vi "FlexMag - 23-03-2023.vi"() -> ()   [LabVIEW 2018] (continued)
                                }
                                frame #1 {
                                n20432 = local read "abort ch2"() -> (w24637:bool)
                                n20433 = case shown="False" w24637 {
                                frame False {
                                n20434 = local read "coating start"() -> (w24638:bool)
                                n20435 = case shown="True" w24638 {
                                frame False {
                                }
                                frame True {
                                n20436 = while {
                                i -> [w24644]
                                stop <- w24646 stop-if-true
                                n20437 = Greater Or Equal?(x=w24644, y=50) -> (x >= y?=w24645:bool)
                                n20438 = case shown="True" w24645 {
                                frame False {
                                }
                                frame True {
                                n20439 = local write "Warning Message"("Automatic Coating Process is canceled !\nCH2 Argon Set Zero problem..." ("Warning Message")) -> ()
                                n20440 = local write "coating error"(TRUE ("coating error")) -> ()
                                }
                                }
                                n20441 = local read "ch2 argon mfc actual"() -> (w24640:dbl)
                                n20442 = Less?(x=w24640, y=1.0) -> (x < y?=w24641:bool)
                                n20443 = case shown="False" w24641 {
                                tunnel: [FALSE ("CH2_WFC_DO") TRUE ("CH2_WFC_DO")] -> w24649
                                frame False {
                                n20444 = Wait Until Next ms Multiple(millisecond multiple=u32 1000) -> ()  [unwired: 1 out]
                                n20445 = local write "ch2 ar set zero auto"(TRUE ("coating error")) -> ()
                                }
                                frame True {
                                }
                                }
                                n20446 = local read "coating start"() -> (w24648:bool)
                                n20447 = local read "abort ch2"() -> (w24642:bool)
                                n20448 = Not(x=w24648) -> (.not. x?=w24647:bool)
                                n20449 = Compound Arithmetic op=OR(w24649, w24647, w24642) -> (w24646:bool)
                                }
                                }
                                }
                                }
                                frame True {
                                }
                                }
                                }
                                frame #2 {
                                n20450 = local read "abort ch2"() -> (w24656:bool)
                                n20451 = case shown="False" w24656 {
                                frame False {
                                n20452 = local read "coating start"() -> (w24657:bool)
                                n20453 = case shown="True" w24657 {
                                frame False {
                                }
                                frame True {
                                n20454 = Wait (ms)(milliseconds to wait=u32 100) -> ()  [unwired: 1 out]
                                "coating ch2 led 15" <- TRUE ("coating ch2 led 1")
                                }
                                }
                                }
                                frame True {
                                }
                                }
                                }
                                }
                                }
                                frame #16 {
                                # "Ar SoV close"
                                n20455 = stacked-sequence {
                                frame #0 {
                                n20456 = local read "abort ch2"() -> (w24660:bool)
                                n20457 = case shown="False" w24660 {
                                frame False {
                                n20458 = local read "coating start"() -> (w24661:bool)
                                n20459 = case shown="True" w24661 {
                                frame False {
                                }
                                frame True {
                                n20460 = while {
                                i -> [w24665]
                                stop <- w24667 stop-if-true
                                n20461 = Greater Or Equal?(x=w24665, y=100) -> (x >= y?=w24666:bool)
                                n20462 = case shown="True" w24666 {
                                frame False {
                                }
                                frame True {
                                n20463 = local write "Warning Message"("Automatic Coating Process is canceled !\nCH2 Argon SoV couldn't be closed..." ("Warning Message")) -> ()
                                n20464 = local write "coating error"(TRUE ("coating error")) -> ()
                                }
                                }
                                n20465 = local read "CH2_SoV_Ar_DI"() -> (w24662:bool)
                                n20466 = case shown="True" w24662 {
                                tunnel: [TRUE ("CH2_WFC_DO") FALSE ("CH2_WFC_DO")] -> w24670
                                frame False {
                                }
                                frame True {
                                n20467 = Wait Until Next ms Multiple(millisecond multiple=u32 200) -> ()  [unwired: 1 out]
                                n20468 = local write "CH2_SoV_Ar_DO"(FALSE ("coating error")) -> ()
                                }
                                }
                                n20469 = local read "coating start"() -> (w24669:bool)
                                n20470 = local read "abort ch2"() -> (w24663:bool)
                                n20471 = Not(x=w24669) -> (.not. x?=w24668:bool)
                                n20472 = Compound Arithmetic op=OR(w24670, w24668, w24663) -> (w24667:bool)
                                }
                                }
                                }
                                }
                                frame True {
                                }
                                }
                                }
                                frame #1 {
                                n20473 = local read "abort ch2"() -> (w24677:bool)
                                n20474 = case shown="False" w24677 {
                                frame False {
                                n20475 = local read "coating start"() -> (w24678:bool)
                                n20476 = case shown="True" w24678 {
                                frame False {
                                }
                                frame True {
                                n20477 = Wait (ms)(milliseconds to wait=u32 100) -> ()  [unwired: 1 out]
                                "coating ch2 led 16" <- TRUE ("coating ch2 led 1")
                                }
                                }
                                }
                                frame True {
                                }
                                }
                                }
                                }
                                }
                                frame #17 {
                                # "BG BV close"
                                n20478 = stacked-sequence {
                                frame #0 {
                                n20479 = local read "abort ch2"() -> (w24681:bool)
                                n20480 = case shown="False" w24681 {
                                frame False {
                                n20481 = local read "coating start"() -> (w24682:bool)
                                n20482 = case shown="True" w24682 {
                                frame False {
                                }
                                frame True {
                                n20483 = while {
                                i -> [w24686]
                                stop <- w24688 stop-if-true
                                n20484 = Greater Or Equal?(x=w24686, y=100) -> (x >= y?=w24687:bool)
                                n20485 = case shown="True" w24687 {
                                frame False {
                                }
                                frame True {
                                n20486 = local write "Warning Message"("Automatic Coating Process is canceled !\nCH2 BG BV couldn't be closed..." ("Warning Message")) -> ()
                                n20487 = local write "coating error"(TRUE ("coating error")) -> ()
                                }
                                }
                                n20488 = local read "CH2_BG_BV_DI"() -> (w24683:bool)
                                n20489 = case shown="True" w24683 {
                                tunnel: [TRUE ("CH2_WFC_DO") FALSE ("CH2_WFC_DO")] -> w24691
                                frame False {
                                }
                                frame True {
                                n20490 = Wait Until Next ms Multiple(millisecond multiple=u32 200) -> ()  [unwired: 1 out]
                                n20491 = local write "CH2_BG_BV_DO"(FALSE ("coating error")) -> ()
                                }
                                }
                                n20492 = local read "coating start"() -> (w24690:bool)
                                n20493 = local read "abort ch2"() -> (w24684:bool)
                                n20494 = Not(x=w24690) -> (.not. x?=w24689:bool)
                                n20495 = Compound Arithmetic op=OR(w24691, w24689, w24684) -> (w24688:bool)
                                }
                                }
                                }
                                }
                                frame True {
                                }
                                }
                                }
                                frame #1 {
                                n20496 = local read "abort ch2"() -> (w24698:bool)
                                n20497 = case shown="False" w24698 {
                                frame False {
                                n20498 = local read "coating start"() -> (w24699:bool)
                                n20499 = case shown="True" w24699 {
                                frame False {
                                }
                                frame True {
                                n20500 = Wait (ms)(milliseconds to wait=u32 100) -> ()  [unwired: 1 out]
                                "coating ch2 led 17" <- TRUE ("coating ch2 led 1")
                                }
                                }
                                }
                                frame True {
                                }
                                }
                                }
                                }
                                }
                                frame #18 {
                                # "CC open"
                                n20501 = stacked-sequence {
                                frame #0 {
                                n20502 = local read "abort ch2"() -> (w24702:bool)
                                n20503 = case shown="False" w24702 {
                                frame False {
                                n20504 = local read "coating start"() -> (w24703:bool)
                                n20505 = case shown="True" w24703 {
                                frame False {
                                }
                                frame True {
                                n20506 = while {
                                i -> [w24707]
                                stop <- w24709 stop-if-true
                                n20507 = Greater Or Equal?(x=w24707, y=100) -> (x >= y?=w24708:bool)
                                n20508 = case shown="True" w24708 {
                                frame False {
                                }
                                frame True {
                                n20509 = local write "Warning Message"("Automatic Coating Process is canceled !\nCH2 CC couldn't be opened..." ("Warning Message")) -> ()
                                n20510 = local write "coating error"(TRUE ("coating error")) -> ()
                                }
                                }
                                n20511 = local read "CH2_CC_DI"() -> (w24704:bool)
                                n20512 = case shown="False" w24704 {
                                tunnel: [FALSE ("CH2_WFC_DO") TRUE ("CH2_WFC_DO")] -> w24712
                                frame False {
                                n20513 = Wait Until Next ms Multiple(millisecond multiple=u32 200) -> ()  [unwired: 1 out]
                                n20514 = local write "CH2_CC_DO"(TRUE ("coating error")) -> ()
                                }
                                frame True {
                                }
                                }
                                n20515 = local read "coating start"() -> (w24711:bool)
                                n20516 = local read "abort ch2"() -> (w24705:bool)
                                n20517 = Not(x=w24711) -> (.not. x?=w24710:bool)
                                n20518 = Compound Arithmetic op=OR(w24712, w24710, w24705) -> (w24709:bool)
                                }
                                }
                                }
                                }
                                frame True {
                                }
                                }
                                }
                                frame #1 {
                                n20519 = local read "abort ch2"() -> (w24719:bool)
                                n20520 = case shown="False" w24719 {
                                frame False {
                                n20521 = local read "coating start"() -> (w24720:bool)
                                n20522 = case shown="True" w24720 {
                                frame False {
                                }
                                frame True {
                                n20523 = Wait (ms)(milliseconds to wait=u32 100) -> ()  [unwired: 1 out]
                                "coating ch2 led 18" <- TRUE ("coating ch2 led 1")
                                }
                                }
                                }
                                frame True {
                                }
                                }
                                }
                                }
                                }
                                frame #19 {
                                # "water close"
                                n20524 = stacked-sequence {
                                frame #0 {
                                n20525 = local read "abort ch2"() -> (w24723:bool)
                                n20526 = case shown="False" w24723 {
                                frame False {
                                n20527 = local read "coating start"() -> (w24724:bool)
                                n20528 = case shown="True" w24724 {
                                frame False {
                                }
                                frame True {
                                n20529 = while {
                                i -> [w24728]
                                stop <- w24730 stop-if-true
                                n20530 = Greater Or Equal?(x=w24728, y=100) -> (x >= y?=w24729:bool)
                                n20531 = case shown="True" w24729 {
                                frame False {
                                }
                                frame True {
                                n20532 = local write "Warning Message"("Automatic Coating Process is canceled !\nCH2 Water Flow couldn't be closed..." ("Warning Message")) -> ()
                                n20533 = local write "coating error"(TRUE ("coating error")) -> ()
                                }
                                }
                                n20534 = local read "CH2_WFC_DI"() -> (w24725:bool)
                                n20535 = case shown="True" w24725 {
                                tunnel: [TRUE ("CH2_WFC_DO") FALSE ("CH2_WFC_DO")] -> w24733
                                frame False {
                                }
                                frame True {
                                n20536 = Wait Until Next ms Multiple(millisecond multiple=u32 200) -> ()  [unwired: 1 out]
                                n20537 = local write "CH2_WFC_DO"(FALSE ("coating error")) -> ()
                                }
                                }
                                n20538 = local read "coating start"() -> (w24732:bool)
                                n20539 = local read "abort ch2"() -> (w24726:bool)
                                n20540 = Not(x=w24732) -> (.not. x?=w24731:bool)
                                n20541 = Compound Arithmetic op=OR(w24733, w24731, w24726) -> (w24730:bool)
                                }
                                }
                                }
                                }
                                frame True {
                                }
                                }
                                }
                                frame #1 {
                                n20542 = local read "abort ch2"() -> (w24740:bool)
                                n20543 = case shown="False" w24740 {
                                frame False {
                                n20544 = local read "coating start"() -> (w24741:bool)
                                n20545 = case shown="True" w24741 {
                                frame False {
                                }
                                frame True {
                                n20546 = Wait (ms)(milliseconds to wait=u32 100) -> ()  [unwired: 1 out]
                                "coating ch2 led 19" <- TRUE ("coating ch2 led 1")
                                }
                                }
                                }
                                frame True {
                                }
                                }
                                }
                                }
                                }
                                frame #20 {
                                # "back roll"
                                n20547 = stacked-sequence {
                                frame #0 {
                                n20548 = local read "abort ch2"() -> (w24744:bool)
                                n20549 = case shown="False" w24744 {
                                frame False {
                                n20550 = local read "coating start"() -> (w24745:bool)
                                n20551 = case shown="True" w24745 {
                                frame False {
                                }
                                frame True {
                                n20552 = disable-structure shown="Enabled" {
                                frame Disabled {
                                n20553 = flat-sequence {
                                frame #0 {
                                n20554 = local read "R DC number steps"() -> (w24746:dbl)
                                n20555 = local write "step count"(w24746) -> ()
                                n20556 = local write "back roll"(TRUE ("back roll")) -> ()
                                }
                                frame #1 {
                                n20557 = Wait (ms)(milliseconds to wait=u32 1000) -> ()  [unwired: 1 out]
                                }
                                frame #2 {
                                n20558 = while {
                                i -> [w24750]
                                stop <- w24757 stop-if-true
                                n20559 = local read "coating start"() -> (w24754:bool)
                                n20560 = local read "back roll"() -> (w24753:bool)
                                n20561 = local read "abort ch2"() -> (w24756:bool)
                                n20562 = Greater?(x=w24750, y=2000) -> (0:w24749:bool)
                                n20563 = Not(x=w24753) -> (.not. x?=w24752:bool)
                                n20564 = Not(x=w24754) -> (.not. x?=w24758:bool)
                                n20565 = local write "coating error"(w24749) -> ()
                                n20566 = Compound Arithmetic op=OR(w24752, w24758, w24756) -> (w24757:bool)
                                n20567 = Wait Until Next ms Multiple(millisecond multiple=u32 200) -> ()  [unwired: 1 out]
                                }
                                }
                                }
                                }
                                frame Enabled {
                                n20568 = local read "dep. for?"() -> (w24760:bool)
                                n20569 = Not(x=w24760) -> (.not. x?=w24761:bool)
                                n20570 = Wait (ms)(milliseconds to wait=u32 100) -> ()  [unwired: 1 out]
                                n20571 = local write "dep. for?"(w24761) -> ()
                                }
                                }
                                }
                                }
                                }
                                frame True {
                                }
                                }
                                }
                                frame #1 {
                                n20572 = local read "abort ch2"() -> (w24762:bool)
                                n20573 = case shown="False" w24762 {
                                frame False {
                                n20574 = local read "coating start"() -> (w24763:bool)
                                n20575 = case shown="True" w24763 {
                                frame False {
                                }
                                frame True {
                                n20576 = Wait (ms)(milliseconds to wait=u32 100) -> ()  [unwired: 1 out]
                                "coating ch2 led 20" <- TRUE ("coating ch2 led 1")
                                }
                                }
                                }
                                frame True {
                                }
                                }
                                }
                                }
                                }
                                frame #21 {
                                # "done"
                                n20577 = stacked-sequence {
                                frame #0 {
                                n20578 = local read "abort ch2"() -> (w24766:bool)
                                n20579 = case shown="False" w24766 {
                                frame False {
                                n20580 = local read "coating start"() -> (w24767:bool)
                                n20581 = case shown="True" w24767 {
                                frame False {
                                }
                                frame True {
                                n20582 = local write "Buzzer DO"(TRUE ("Buzzer DO")) -> ()
                                n20583 = Wait (ms)(milliseconds to wait=u32 3000) -> ()  [unwired: 1 out]
                                n20584 = local write "System Status"("COATING PROCESS DONE (CH2)" ("System Status")) -> ()
                                }
                                }
                                }
                                frame True {
                                }
                                }
                                }
                                frame #1 {
                                n20585 = local read "abort ch2"() -> (w24771:bool)
                                n20586 = case shown="False" w24771 {
                                frame False {
                                n20587 = local read "coating start"() -> (w24772:bool)
                                n20588 = case shown="True" w24772 {
                                frame False {
                                }
                                frame True {
                                n20589 = Wait (ms)(milliseconds to wait=u32 1000) -> ()  [unwired: 1 out]
                                n20590 = local write "System Status"("SEMI-AUTOMATIC MODE " ("System Status")) -> ()
                                n20591 = local write "Buzzer DO"(FALSE ("Buzzer DO")) -> ()
                                }
                                }
                                }
                                frame True {
                                }
                                }
                                }
                                }
                                }
                                }
                                }
                                }
                                }
                                frame "chamber III" {
                                # "CH III"
                                n20592 = disable-structure shown="Disabled" {
                                disable-tunnel: [w24783 TRUE] -> w24776
                                frame Disabled {
                                n20593 = local read "ch3 cc torr"() -> (w24779:dbl)
                                n20594 = local read "ch3 ch pg torr"() -> (w24782:dbl)
                                n20595 = Less Or Equal?(x=w24782, y=0.005) -> (x <= y?=w24780:bool)
                                n20596 = Less Or Equal?(x=w24779, y=0.005) -> (x <= y?=w24781:bool)
                                n20597 = And(x=w24780, y=w24781) -> (x .and. y?=w24783:bool)
                                }
                                frame Enabled {
                                }
                                }
                                n20598 = case shown="True" w24776 {
                                frame False {
                                n20599 = local write "coating error"(TRUE ("coating error")) -> ()
                                n20600 = local write "Warning Message"("Automatic Coating Process is canceled !\nCH3 Pressure should be under 5E-3 Torr .." ("Warning Message")) -> ()
                                }
                                frame True {
                                n20601 = stacked-sequence {
                                frame #0 {
                                }
                                frame #1 {
                                n20602 = stacked-sequence {
                                frame #0 {
                                n20603 = local read "abort ch3"() -> (w24787:bool)
                                n20604 = case shown="False" w24787 {
                                frame False {
                                n20605 = local read "coating start"() -> (w24788:bool)
                                n20606 = case shown="True" w24788 {
                                frame False {
                                }
                                frame True {
                                n20607 = local read "casette_ch3_gui"() -> (w24790:bool)
                                n20608 = Wait (ms)(milliseconds to wait=u32 100) -> ()  [unwired: 1 out]
                                n20609 = case shown="False" w24790 {
                                frame False {
                                n20610 = stacked-sequence {
                                frame #0 {
                                n20611 = flat-sequence {
                                frame #0 {
                                n20612 = local write "target chamber"(3.0 ("target chamber")) -> ()
                                n20613 = Wait (ms)(milliseconds to wait=u32 100) -> ()  [unwired: 1 out]
                                }
                                frame #1 {
                                n20614 = Wait (ms)(milliseconds to wait=u32 1000) -> ()  [unwired: 1 out]
                                }
                                frame #2 {
                                n20615 = local write "transfer vacuum auto"(TRUE ("transfer vacuum")) -> ()
                                }
                                }
                                }
                                frame #1 {
                                n20616 = while {
                                i -> [w24798]
                                stop <- w24800 stop-if-true
                                # "20min"
                                n20617 = local read "present location"() -> (w24804:dbl)
                                n20618 = local read "casette_ch3_gui"() -> (w24796:bool)
                                n20619 = local read "abort ch3"() -> (w24799:bool)
                                n20620 = Equal?(x=w24804, y=3.0) -> (x = y?=w24802:bool)
                                n20621 = Greater?(x=w24798, y=1200) -> (0:w24795:bool)
                                n20622 = Compound Arithmetic op=OR(w24799, w24802, w24796, w24795) -> (w24800:bool)
                                n20623 = local write "trns error"(w24795) -> ()
                                n20624 = Wait Until Next ms Multiple(millisecond multiple=u32 1000) -> ()  [unwired: 1 out]
                                }
                                }
                                }
                                }
                                frame True {
                                }
                                }
                                }
                                }
                                }
                                frame True {
                                }
                                }
                                }
                                frame #1 {
                                n20625 = local read "abort ch3"() -> (w24805:bool)
                                n20626 = case shown="False" w24805 {
                                frame False {
                                n20627 = local read "coating start"() -> (w24806:bool)
                                n20628 = case shown="True" w24806 {
                                frame False {
                                }
                                frame True {
                                n20629 = Wait (ms)(milliseconds to wait=u32 100) -> ()  [unwired: 1 out]
                                n20630 = local write "System Status"("COATING MODE ACTIVE" ("System Status")) -> ()
                                "coating ch3 led 1" <- TRUE ("coating ch2 led 1")
                                }
                                }
                                }
                                frame True {
                                }
                                }
                                }
                                }
                                }
                                frame #2 {
                                # "water"
                                n20631 = stacked-sequence {
                                frame #0 {
                                # "ch1 water off"
                                n20632 = local read "abort ch3"() -> (w24810:bool)
                                n20633 = case shown="False" w24810 {
                                frame False {
                                n20634 = local read "coating start"() -> (w24811:bool)
                                n20635 = case shown="True" w24811 {
                                frame False {
                                }
                                frame True {
                                n20636 = while {
                                i -> [w24814]
                                stop <- w24816 stop-if-true
                                n20637 = Greater Or Equal?(x=w24814, y=100) -> (x >= y?=w24815:bool)
                                n20638 = case shown="True" w24815 {
                                frame False {
                                }
                                frame True {
                                n20639 = local write "coating error"(TRUE ("coating error")) -> ()
                                n20640 = local write "Warning Message"("Automatic Coating Process is canceled !\nCH1 Water Flow Problem.." ("Warning Message")) -> ()
                                }
                                }
                                n20641 = local read "CH1_WFC_DI"() -> (w24820:bool)
                                n20642 = case shown="True" w24820 {
                                tunnel: [TRUE ("CH2_WFC_DO") FALSE ("CH2_WFC_DO")] -> w24819
                                frame False {
                                }
                                frame True {
                                n20643 = Wait Until Next ms Multiple(millisecond multiple=u32 200) -> ()  [unwired: 1 out]
                                n20644 = local write "CH1_WFC_DO"(FALSE ("CH2_WFC_DO")) -> ()
                                }
                                }
                                n20645 = local read "coating start"() -> (w24818:bool)
                                n20646 = local read "abort ch3"() -> (w24812:bool)
                                n20647 = Not(x=w24818) -> (.not. x?=w24817:bool)
                                n20648 = Compound Arithmetic op=OR(w24819, w24817, w24812) -> (w24816:bool)
                                }
                                }
                                }
                                }
                                frame True {
                                }
                                }
                                }
                                frame #1 {
                                # "ch2 water off"
                                n20649 = local read "abort ch3"() -> (w24827:bool)
                                n20650 = case shown="False" w24827 {
                                frame False {
                                n20651 = local read "coating start"() -> (w24828:bool)
                                n20652 = case shown="True" w24828 {
                                frame False {
                                }
                                frame True {
                                n20653 = while {
                                i -> [w24831]
                                stop <- w24833 stop-if-true
                                n20654 = Greater Or Equal?(x=w24831, y=100) -> (x >= y?=w24832:bool)
                                n20655 = case shown="True" w24832 {
                                frame False {
                                }
                                frame True {
                                n20656 = local write "coating error"(TRUE ("coating error")) -> ()
                                n20657 = local write "Warning Message"("Automatic Coating Process is canceled !\nCH2 Water Flow Problem.." ("Warning Message")) -> ()
                                }
                                }
                                n20658 = local read "CH2_WFC_DI"() -> (w24837:bool)
                                n20659 = case shown="True" w24837 {
                                tunnel: [TRUE ("CH2_WFC_DO") FALSE ("CH2_WFC_DO")] -> w24836
                                frame False {
                                }
                                frame True {
                                n20660 = Wait Until Next ms Multiple(millisecond multiple=u32 200) -> ()  [unwired: 1 out]
                                n20661 = local write "CH2_WFC_DO"(FALSE ("CH2_WFC_DO")) -> ()
                                }
                                }
                                n20662 = local read "coating start"() -> (w24835:bool)
                                n20663 = local read "abort ch3"() -> (w24829:bool)
                                n20664 = Not(x=w24835) -> (.not. x?=w24834:bool)
                                n20665 = Compound Arithmetic op=OR(w24836, w24834, w24829) -> (w24833:bool)
                                }
                                }
                                }
                                }
                                frame True {
                                }
                                }
                                }
                                frame #2 {
                                # "ch4 water off"
                                n20666 = local read "abort ch3"() -> (w24844:bool)
                                n20667 = case shown="False" w24844 {
                                frame False {
                                n20668 = local read "coating start"() -> (w24845:bool)
                                n20669 = case shown="True" w24845 {
                                frame False {
                                }
                                frame True {
                                n20670 = while {
                                i -> [w24848]
                                stop <- w24850 stop-if-true
                                n20671 = Greater Or Equal?(x=w24848, y=100) -> (x >= y?=w24849:bool)
                                n20672 = case shown="True" w24849 {
                                frame False {
                                }
                                frame True {
                                n20673 = local write "coating error"(TRUE ("coating error")) -> ()
                                n20674 = local write "Warning Message"("Automatic Coating Process is canceled !\nCH4 Water Flow Problem.." ("Warning Message")) -> ()
                                }
                                }
                                n20675 = local read "CH4_WFC_DI"() -> (w24854:bool)
                                n20676 = case shown="True" w24854 {
                                tunnel: [TRUE ("CH2_WFC_DO") FALSE ("CH2_WFC_DO")] -> w24853
                                frame False {
                                }
                                frame True {
                                n20677 = Wait Until Next ms Multiple(millisecond multiple=u32 200) -> ()  [unwired: 1 out]
                                n20678 = local write "CH4_WFC_DO"(FALSE ("CH2_WFC_DO")) -> ()
                                }
                                }
                                n20679 = local read "coating start"() -> (w24852:bool)
                                n20680 = local read "abort ch3"() -> (w24846:bool)
                                n20681 = Not(x=w24852) -> (.not. x?=w24851:bool)
                                n20682 = Compound Arithmetic op=OR(w24853, w24851, w24846) -> (w24850:bool)
                                }
                                }
                                }
                                }
                                frame True {
                                }
                                }
                                }
                                frame #3 {
                                # "ch3 water on"
                                n20683 = local read "abort ch3"() -> (w24861:bool)
                                n20684 = case shown="False" w24861 {
                                frame False {
                                n20685 = local read "coating start"() -> (w24862:bool)
                                n20686 = case shown="True" w24862 {
                                frame False {
                                }
                                frame True {
                                n20687 = while {
                                i -> [w24865]
                                stop <- w24867 stop-if-true
                                n20688 = Greater Or Equal?(x=w24865, y=100) -> (x >= y?=w24866:bool)
                                n20689 = case shown="True" w24866 {
                                frame False {
                                }
                                frame True {
                                n20690 = local write "coating error"(TRUE ("coating error")) -> ()
                                n20691 = local write "Warning Message"("Automatic Coating Process is canceled !\nCH3 Water Flow Problem.." ("Warning Message")) -> ()
                                }
                                }
                                n20692 = local read "CH3_WFC_DI"() -> (w24871:bool)
                                n20693 = case shown="False" w24871 {
                                tunnel: [FALSE ("CH2_WFC_DO") TRUE ("CH2_WFC_DO")] -> w24870
                                frame False {
                                n20694 = Wait Until Next ms Multiple(millisecond multiple=u32 200) -> ()  [unwired: 1 out]
                                n20695 = local write "CH3_WFC_DO"(TRUE ("CH2_WFC_DO")) -> ()
                                }
                                frame True {
                                }
                                }
                                n20696 = local read "coating start"() -> (w24869:bool)
                                n20697 = local read "abort ch3"() -> (w24863:bool)
                                n20698 = Not(x=w24869) -> (.not. x?=w24868:bool)
                                n20699 = Compound Arithmetic op=OR(w24870, w24868, w24863) -> (w24867:bool)
                                }
                                }
                                }
                                }
                                frame True {
                                }
                                }
                                }
                                frame #4 {
                                n20700 = local read "abort ch3"() -> (w24878:bool)
                                n20701 = case shown="False" w24878 {
                                frame False {
                                n20702 = local read "coating start"() -> (w24879:bool)
                                n20703 = case shown="True" w24879 {
                                frame False {
                                }
                                frame True {
                                n20704 = Wait (ms)(milliseconds to wait=u32 100) -> ()  [unwired: 1 out]
                                "coating ch3 led 2" <- TRUE ("coating ch2 led 1")
                                }
                                }
                                }
                                frame True {
                                }
                                }
                                }
                                }
                                }
                                frame #3 {
                                # "ch3 pcgv on"
                                n20705 = stacked-sequence {
                                frame #0 {
                                n20706 = local read "abort ch3"() -> (w24882:bool)
                                n20707 = case shown="False" w24882 {
                                frame False {
                                n20708 = local read "coating start"() -> (w24883:bool)
                                n20709 = case shown="True" w24883 {
                                frame False {
                                }
                                frame True {
                                n20710 = local read "ch3_pcgv_gui"() -> (w24884:bool)
                                n20711 = case shown="False" w24884 {
                                frame False {
                                n20712 = flat-sequence {
                                frame #0 {
                                n20713 = local write "pcgv3 auto open"(TRUE ("pcgv2 auto open")) -> ()
                                }
                                frame #1 {
                                n20714 = Wait (ms)(milliseconds to wait=u32 1000) -> ()  [unwired: 1 out]
                                }
                                frame #2 {
                                n20715 = local write "pcgv3 auto open"(TRUE ("pcgv2 auto open")) -> ()
                                }
                                }
                                }
                                frame True {
                                }
                                }
                                }
                                }
                                }
                                frame True {
                                }
                                }
                                }
                                frame #1 {
                                n20716 = local read "abort ch3"() -> (w24888:bool)
                                n20717 = case shown="False" w24888 {
                                frame False {
                                n20718 = local read "coating start"() -> (w24889:bool)
                                n20719 = case shown="True" w24889 {
                                frame False {
                                }
                                frame True {
                                n20720 = while {
                                i -> [w24892]
                                stop <- w24894 stop-if-true
                                n20721 = Greater Or Equal?(x=w24892, y=100) -> (x >= y?=w24893:bool)
                                n20722 = case shown="True" w24893 {
                                frame False {
                                }
                                frame True {
                                n20723 = local write "coating error"(TRUE ("coating error")) -> ()
                                n20724 = local write "Warning Message"("Automatic Coating Process is canceled !\nCH3 PCGV couldn't be opened.." ("Warning Message")) -> ()
                                }
                                }
                                n20725 = local read "ch3_pcgv_gui"() -> (w24898:bool)
                                n20726 = case shown="False" w24898 {
                                tunnel: [FALSE ("CH2_WFC_DO") TRUE ("CH2_WFC_DO")] -> w24897
                                frame False {
                                n20727 = Wait Until Next ms Multiple(millisecond multiple=u32 200) -> ()  [unwired: 1 out]
                                }
                                frame True {
                                }
                                }
                                n20728 = local read "coating start"() -> (w24896:bool)
                                n20729 = local read "abort ch3"() -> (w24890:bool)
                                n20730 = Not(x=w24896) -> (.not. x?=w24895:bool)
                                n20731 = Compound Arithmetic op=OR(w24897, w24895, w24890) -> (w24894:bool)
                                }
                                }
                                }
                                }
                                frame True {
                                }
                                }
                                }
                                frame #2 {
                                n20732 = local read "abort ch3"() -> (w24904:bool)
                                n20733 = case shown="False" w24904 {
                                frame False {
                                n20734 = local read "coating start"() -> (w24905:bool)
                                n20735 = case shown="True" w24905 {
                                frame False {
                                }
                                frame True {
                                n20736 = Wait (ms)(milliseconds to wait=u32 100) -> ()  [unwired: 1 out]
                                "coating ch3 led 3" <- TRUE ("coating ch2 led 1")
                                }
                                }
                                }
                                frame True {
                                }
                                }
                                }
                                }
                                }
                                frame #4 {
                                # "DC host - communication check"
                                n20737 = stacked-sequence {
                                frame #0 {
                                n20738 = local read "abort ch3"() -> (w24908:bool)
                                n20739 = case shown="False" w24908 {
                                frame False {
                                n20740 = local read "coating start"() -> (w24909:bool)
                                n20741 = case shown="True" w24909 {
                                frame False {
                                }
                                frame True {
                                n20742 = flat-sequence {
                                frame #0 {
                                n20743 = local write "Dc_host_auto"(TRUE ("pcgv2 auto open")) -> ()
                                }
                                frame #1 {
                                n20744 = Wait (ms)(milliseconds to wait=u32 1000) -> ()  [unwired: 1 out]
                                }
                                frame #2 {
                                n20745 = local write "Dc_host_auto"(TRUE ("pcgv2 auto open")) -> ()
                                }
                                }
                                }
                                }
                                }
                                frame True {
                                }
                                }
                                }
                                frame #1 {
                                n20746 = local read "abort ch3"() -> (w24913:bool)
                                n20747 = case shown="False" w24913 {
                                frame False {
                                n20748 = local read "coating start"() -> (w24914:bool)
                                n20749 = case shown="True" w24914 {
                                frame False {
                                }
                                frame True {
                                n20750 = while {
                                i -> [w24917]
                                stop <- w24919 stop-if-true
                                n20751 = Greater Or Equal?(x=w24917, y=100) -> (x >= y?=w24918:bool)
                                n20752 = case shown="True" w24918 {
                                frame False {
                                }
                                frame True {
                                n20753 = local write "coating error"(TRUE ("coating error")) -> ()
                                n20754 = local write "Warning Message"("Automatic Coating Process is canceled !\nDCPS Problem.." ("Warning Message")) -> ()
                                }
                                }
                                n20755 = local read "Dcps_fail"() -> (w24923:bool)
                                n20756 = case shown="True" w24923 {
                                tunnel: [TRUE ("CH2_WFC_DO") FALSE ("CH2_WFC_DO")] -> w24922
                                frame False {
                                }
                                frame True {
                                n20757 = Wait Until Next ms Multiple(millisecond multiple=u32 200) -> ()  [unwired: 1 out]
                                }
                                }
                                n20758 = local read "coating start"() -> (w24921:bool)
                                n20759 = local read "abort ch3"() -> (w24915:bool)
                                n20760 = Not(x=w24921) -> (.not. x?=w24920:bool)
                                n20761 = Compound Arithmetic op=OR(w24922, w24920, w24915) -> (w24919:bool)
                                }
                                }
                                }
                                }
                                frame True {
                                }
                                }
                                }
                                frame #2 {
                                n20762 = local read "abort ch3"() -> (w24929:bool)
                                n20763 = case shown="False" w24929 {
                                frame False {
                                n20764 = local read "coating start"() -> (w24930:bool)
                                n20765 = case shown="True" w24930 {
                                frame False {
                                }
                                frame True {
                                n20766 = Wait (ms)(milliseconds to wait=u32 100) -> ()  [unwired: 1 out]
                                "coating ch3 led 4" <- TRUE ("coating ch2 led 1")
                                }
                                }
                                }
                                frame True {
                                }
                                }
                                }
                                }
                                }
                                frame #5 {
                                # "magnetron selection"
                                n20767 = stacked-sequence {
                                frame #0 {
                                n20768 = local read "abort ch3"() -> (w24933:bool)
                                n20769 = case shown="False" w24933 {
                                frame False {
                                n20770 = local read "coating start"() -> (w24934:bool)
                                n20771 = case shown="True" w24934 {
                                frame False {
                                }
                                frame True {
                                n20772 = local write "DCPS_ SW2 DO"(TRUE ("pcgv2 auto open")) -> ()
                                n20773 = local write "DCPS_ SW1 DO"(FALSE ("pcgv2 auto open")) -> ()
                                n20774 = Wait (ms)(milliseconds to wait=u32 1000) -> ()  [unwired: 1 out]
                                }
                                }
                                }
                                frame True {
                                }
                                }
                                }
                                frame #1 {
                                n20775 = local read "abort ch3"() -> (w24938:bool)
                                n20776 = case shown="False" w24938 {
                                frame False {
                                n20777 = local read "coating start"() -> (w24939:bool)
                                n20778 = case shown="True" w24939 {
                                frame False {
                                }
                                frame True {
                                n20779 = while {
                                i -> [w24942]
                                stop <- w24944 stop-if-true
                                n20780 = Greater Or Equal?(x=w24942, y=100) -> (x >= y?=w24943:bool)
                                n20781 = case shown="True" w24943 {
                                frame False {
                                }
                                frame True {
                                n20782 = local write "Warning Message"("Automatic Coating Process is canceled !\nDCPS Magnetron Selection Problem.." ("Warning Message")) -> ()
                                n20783 = local write "coating error"(TRUE ("coating error")) -> ()
                                }
                                }
                                n20784 = local read "DCPS_ SW2 DI"() -> (w24948:bool)
                                n20785 = case shown="False" w24948 {
                                tunnel: [FALSE ("CH2_WFC_DO") TRUE ("CH2_WFC_DO")] -> w24947
                                frame False {
                                n20786 = local write "DCPS_ SW1 DO"(FALSE ("CH2_WFC_DO")) -> ()
                                n20787 = local write "DCPS_ SW2 DO"(TRUE ("CH2_WFC_DO")) -> ()
                                n20788 = Wait Until Next ms Multiple(millisecond multiple=u32 200) -> ()  [unwired: 1 out]
                                }